vi "HFRR ADV v038 new software.vi"() -> ()   [LabVIEW 2025] (continued)
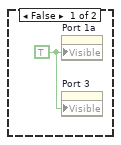
[diagram p5: hidden frame]
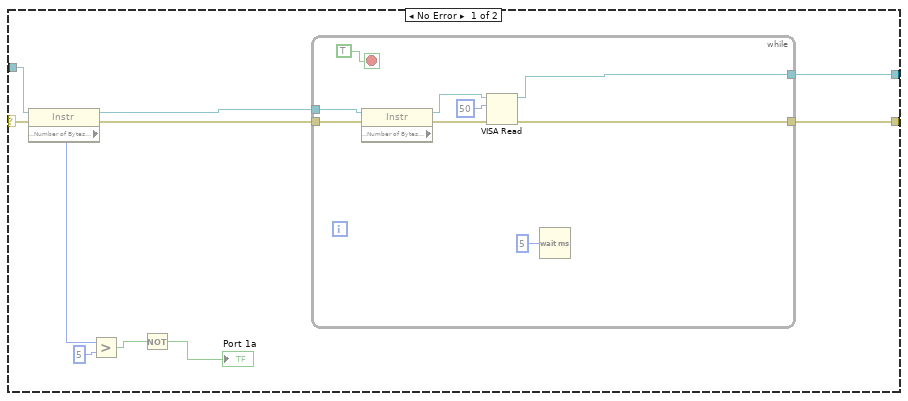
[diagram p6: hidden frame]
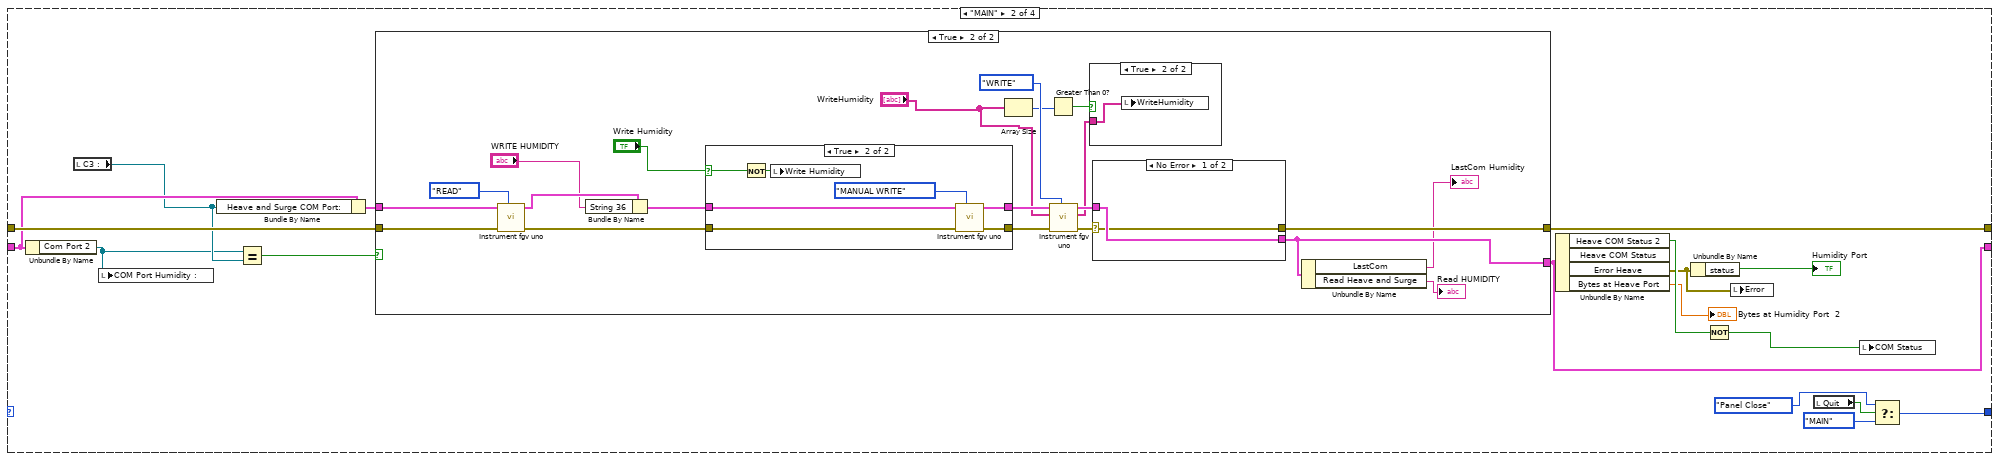
[diagram p9: hidden frame]
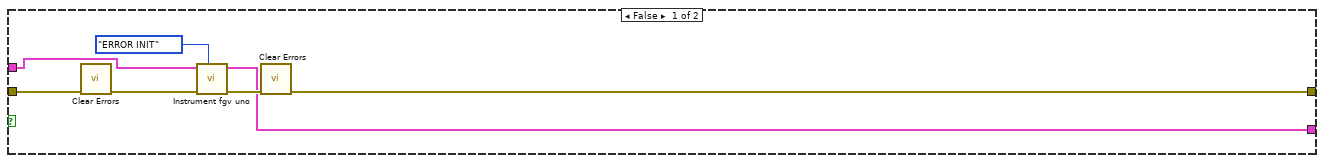
[diagram p10: hidden frame]
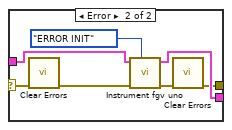
[diagram p12: hidden frame]
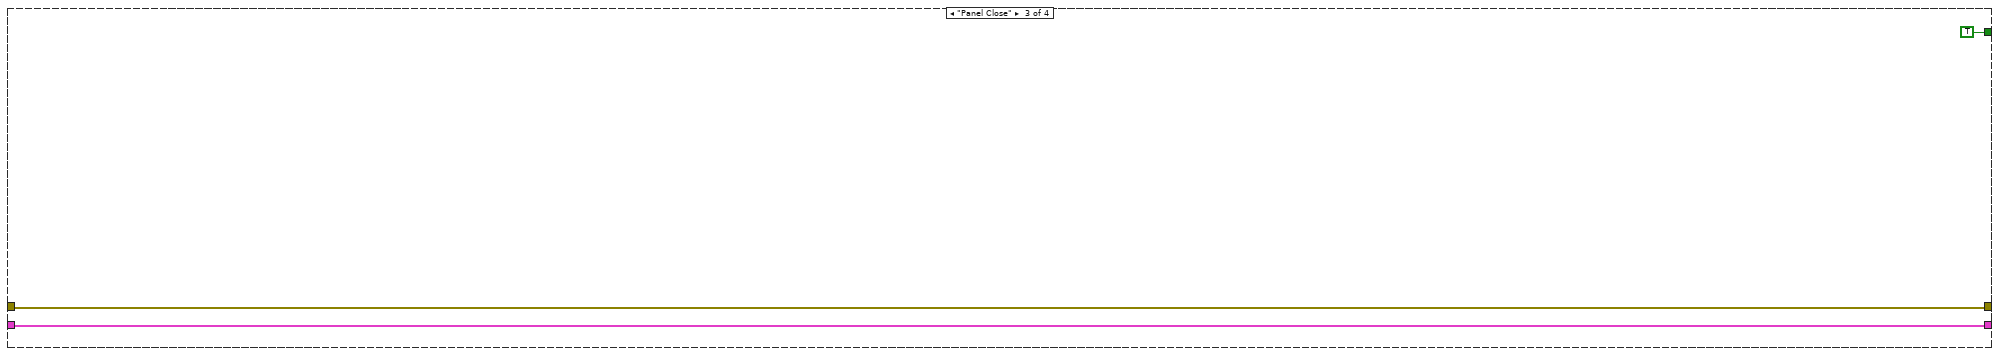
[diagram p14: hidden frame]
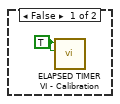
[diagram p18: hidden frame]
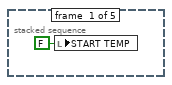
[diagram p20: hidden frame]
        "output Vpp" <- w4065
        n3087 = Number To Fractional String(number=w4065, precision (6)=i16 1) -> (F-format string=w4063:string)  [unwired: 2 in]
        n3088 = Concatenate Strings("DAC;" ("string"), w4063) -> (w4047:string)
        n3089 = local write "Due Write"(w4047) -> ()
        "prev_error" <- w4050
        "integral_accumulator_in" <- w4049
        "prev_vc_cmd" <- w4048
      }
    }
    n3090 = local read "Quit"() -> (w4040:bool)
  }
  n3091 = Or(x=w45, y=w44) -> (x .or. y?=w46:bool)
  n3092 = Or(x=w42, y=w46) -> (x .or. y?=w51:bool)
  n3093 = control-ref of="new picture"() -> ()  [unwired: 1 out]
  n3094 = Or(x=w54, y=w51) -> (x .or. y?=w48:bool)
  n3095 = Or(x=w48, y=w49) -> (x .or. y?=w43:bool)
  n3096 = while {
    tunnel: [w4070] -> w53
    i -> [w4077]
    stop <- w4070 stop-if-true
    n3097 = local read "Quit"() -> (w4070:bool)
    n3098 = Equal To 0?(x=w4077) -> (x = 0?=w4075:bool)
    n3099 = call "Elapsed Time3"("Time Target (s)"=45.0, "Auto Reset"=TRUE) -> ("Time has Elapsed"=w4074:bool)  [unwired: 10 in, 7 out]
    n3100 = Wait (ms)(milliseconds to wait=u32 50) -> ()  [unwired: 1 out]
    n3101 = Or(x=w4074, y=w4075) -> (x .or. y?=w4076:bool)
    n3102 = case shown="True" w4076 {
      frame False {
      }
      frame True {
        n3103 = call <vilib>:"System Exec.vi"("run minimized? (F)"=TRUE, "error in (no error)"="error in (no error)", "command line"="powercfg.exe -change -monitor-timeout-ac 0") -> ("error out"=w4088:errorcluster)  [unwired: 5 in, 3 out]
        n3104 = call <vilib>:"System Exec.vi"("run minimized? (F)"=TRUE, "error in (no error)"=w4088, "command line"="powercfg.exe -change -disk-timeout-ac 0") -> ("error out"=w4087:errorcluster)  [unwired: 5 in, 3 out]
        n3105 = call <vilib>:"System Exec.vi"("run minimized? (F)"=TRUE, "error in (no error)"=w4087, "command line"="powercfg.exe -change -standby-timeout-ac 0") -> ("error out"=w4086:errorcluster)  [unwired: 5 in, 3 out]
        n3106 = call <vilib>:"System Exec.vi"("run minimized? (F)"=TRUE, "error in (no error)"=w4086, "command line"="powercfg.exe -change -hibernate-timeout-ac 0") -> ("error out"=w4085:errorcluster)  [unwired: 5 in, 3 out]
        n3107 = call <vilib>:"Simple Error Handler.vi"("error in (no error)"=w4085) -> ("error out"=w4091:errorcluster)  [unwired: 4 in, 4 out]
        n3108 = call <vilib>:"Clear Errors.vi"("error in (no error)"=w4091) -> ("error out"=→"error out":errorcluster)  [unwired: 5 in, 1 out]
      }
    }
  }
  n3109 = Compound Arithmetic op=OR(w56, w43, w53) -> (w55:bool)
  n3110 = flat-sequence {
    tunnel: w55 -> [_]
    tunnel: [w4093] -> w25
    tunnel: w25 -> [_]
    frame #0 {
      n3111 = call "CLOSE CONNECTION.vi"() -> ("error out"=w4093:errorcluster)  [unwired: 11 in]
    }
    frame #1 {
      n3112 = Quit LabVIEW(quit? (T)=TRUE) -> ()
      n3113 = local write "Quit"(FALSE ("EXIT")) -> ()
    }
  }
  n3114 = property on="Heater Button" class="Bool (strict)"("Visible"=TRUE) -> ()  [unwired: 2 in, 2 out]
  n3115 = while {
    tunnel: [w4100] -> _
    i -> [w4100]
    stop <- w4096 stop-if-true
    # "Langauage selection"
    n3116 = Equal?(x="Lan flag", y=22.0) -> ()  [unwired: 1 out]
    n3117 = disable-structure shown="Disabled" {
      frame Disabled {
        n3118 = stacked-sequence {
          frame #0 {
            n3119 = case shown="\"Russian\"" "Language Selection" {
              tunnel: [0 1] -> w4102
              frame "English", Default {
              }
              frame "Russian" {
              }
            }
            n3120 = for {
              N: 130 -> [_]
              tunnel: "Table" -> [w4111]
              tunnel: w4102 -> [w4110]
              i -> [w4109]
              n3121 = Index Array(array=w4111, index (row)=w4109, index (col)=w4110) -> (element=w4108:string)
              n3122 = case shown="1" w4109 {
                tunnel: w4108 -> [w4112 w4113 _ w4114 w4115 w4116 w4117 w4118 w4119 w4120 w4121 w4122 w4123 w4124 w4125 w4126 w4127 w4128 w4129 w4130 w4131 w4132 w4133 w4134 w4135 w4136 w4137 w4138 w4139 _ _ w4140 w4141 w4142 w4143 w4144 w4145 w4154 w4161 w4168 w4175 w4179 w4182 w4185 w4187 w4189 w4190 w4191 w4192 w4193 w4194 w4195 w4196 w4197 w4198 w4199 w4200 w4201 w4202 w4203 w4204 w4205 w4206 w4207 w4208 w4209 w4210 w4211 w4212 w4213 w4214 w4215 w4216 w4217 w4218 w4219 w4220 w4221 w4222 w4223 w4224 w4225 w4226 w4227 w4228 w4229 w4230 w4231 w4232 w4233 w4234 w4235 w4236 w4237 w4238 w4239 w4240 w4241 w4242 w4243 w4244 w4245 w4246 w4247 w4248 _ w4249 w4250 w4251 w4252 w4253 w4254 w4255 w4256 w4257 w4258 w4259 w4260 w4261 _ w4262 w4263 w4264 w4265 w4266 w4267 _]
                frame 0 {
                  n3123 = local write "S"(w4112) -> ()
                }
                frame 1 {
                  n3124 = local write "S 2"(w4113) -> ()
                }
                frame 2 {
                }
                frame 3 {
                  n3125 = local write "S 4"(w4114) -> ()
                }
                frame 4 {
                  n3126 = property on="FILE" class="Str"("Caption.Text"=w4115) -> ()  [unwired: 2 in, 2 out]
                }
                frame 5 {
                  n3127 = property on="Fuel Discription :" class="Str"("Caption.Text"=w4116) -> ()  [unwired: 2 in, 2 out]
                }
                frame 6 {
                  n3128 = property on="Remarks :" class="Str"("Caption.Text"=w4117) -> ()  [unwired: 2 in, 2 out]
                }
                frame 7 {
                  n3129 = property on="Save & Continue" class="Bool (strict)"("Boolean Text.Text"=w4118) -> ()  [unwired: 2 in, 2 out]
                }
                frame 8 {
                }
                frame 9 {
                  n3130 = property on="Set Hz" class="DigNum (strict)"("Caption.Text"=w4120) -> ()  [unwired: 2 in, 2 out]
                }
                frame 10 {
                }
                frame 11 {
                  n3131 = property on="NORMAL LOAD" class="DigNum (strict)"("Caption.Text"=w4122) -> ()  [unwired: 2 in, 2 out]
                }
                frame 12 {
                }
                frame 13 {
                  n3132 = property on="Set Temp" class="DigNum (strict)"("Caption.Text"=w4124) -> ()  [unwired: 2 in, 2 out]
                }
                frame 14 {
                  n3133 = local write "S 15"(w4125) -> ()
                }
                frame 15 {
                  n3134 = property on="Set Rh" class="DigNum (strict)"("Caption.Text"=w4126) -> ()  [unwired: 2 in, 2 out]
                }
                frame 16 {
                }
                frame 17 {
                  n3135 = local write "S 18"(w4128) -> ()
                }
                frame 18 {
                  "String 17" <- w4129
                }
                frame 19 {
                  n3136 = property on="test time" class="DigNum (strict)"("Caption.Text"=w4130) -> ()  [unwired: 2 in, 2 out]
                }
                frame 20 {
                  "String 18" <- w4131
                  "String 22" <- w4131
                }
                frame 21 {
                  n3137 = property on="Elapsed time" class="DigNum (strict)"("Caption.Text"=w4132) -> ()  [unwired: 2 in, 2 out]
                }
                frame 22 {
                  n3138 = property on="Samplingtime 2" class="DigNum (strict)"("Caption.Text"=w4133) -> ()  [unwired: 2 in, 2 out]
                }
                frame 23 {
                  "String 21" <- w4134
                }
                frame 24 {
                  n3139 = property on="Countdown" class="DigNum (strict)"("Caption.Text"=w4135) -> ()  [unwired: 2 in, 2 out]
                }
                frame 25 {
                  n3140 = property on="Countdown 2" class="DigNum (strict)"("Caption.Text"=w4136) -> ()  [unwired: 2 in, 2 out]
                }
                frame 26 {
                  n3141 = property on="Engage" class="Bool (strict)"("Boolean Text.Text"=w4137) -> ()  [unwired: 2 in, 2 out]
                }
                frame 27 {
                  n3142 = property on="Boolean  4" class="Bool (strict)"("Boolean Text.Text"=w4138) -> ()  [unwired: 2 in, 2 out]
                }
                frame 28 {
                  n3143 = property on="Test \nStatus" class="Bool (strict)"("Boolean Text.Text"=w4139) -> ()  [unwired: 2 in, 2 out]
                }
                frame 29 {
                }
                frame 30 {
                }
                frame 31 {
                }
                frame 32 {
                  n3144 = property on="RSTCOF" class="Bool"("Boolean Text.Text"=w4141) -> ()  [unwired: 2 in, 2 out]
                  n3145 = property on="RST FF" class="Bool"("Boolean Text.Text"=w4141) -> ()  [unwired: 2 in, 2 out]
                  n3146 = property on="RST TEMP" class="Bool"("Boolean Text.Text"=w4141) -> ()  [unwired: 2 in, 2 out]
                  n3147 = property on="RSTV1 3" class="Bool"("Boolean Text.Text"=w4141) -> ()  [unwired: 2 in, 2 out]
                  n3148 = property on="rstv2" class="Bool"("Boolean Text.Text"=w4141) -> ()  [unwired: 2 in, 2 out]
                  n3149 = property on="RSTV1 2" class="Bool"("Boolean Text.Text"=w4141) -> ()  [unwired: 2 in, 2 out]
                  n3150 = property on="RST CP" class="Bool"("Boolean Text.Text"=w4141) -> ()  [unwired: 2 in, 2 out]
                }
                frame 33 {
                  "S 61" <- w4142
                }
                frame 34 {
                  "String 23" <- w4143
                }
                frame 35 {
                  n3151 = property on="Rh Before" class="DigNum (strict)"("Caption.Text"=w4144) -> ()  [unwired: 2 in, 2 out]
                }
                frame 36 {
                  n3152 = Match Pattern(string=w4145, regular expression=",") -> (before substring=→"bs":string, after substring=→"as":string)  [unwired: 1 in, 2 out]
                  n3153 = property on="Rh After" class="DigNum (strict)"("Caption.Text"=w4145) -> ()  [unwired: 2 in, 2 out]
                }
                frame 37 {
                  n3154 = Match Pattern(string=w4154, regular expression=",") -> (before substring=w4153:string, after substring=w4152:string)  [unwired: 1 in, 2 out]
                  "bs" <- w4153
                  "as" <- w4152
                  n3155 = Concatenate Strings(w4153, w4152) -> (w4149:string)
                  n3156 = property on="Humidity before test 2" class="DigNum (strict)"("Caption.Text"=w4149) -> ()  [unwired: 2 in, 2 out]
                  n3157 = Concatenate Strings(w4149, "=" ("string")) -> (w4150:string)
                  n3158 = local write "S 38"(w4150) -> ()
                }
                frame 38 {
                  n3159 = Match Pattern(string=w4161, regular expression=",") -> (before substring=w4160:string, after substring=w4159:string)  [unwired: 1 in, 2 out]
                  "bs" <- w4160
                  "as" <- w4159
                  n3160 = Concatenate Strings(w4160, w4159) -> (w4156:string)
                  n3161 = property on="Humidity after test 2" class="DigNum (strict)"("Caption.Text"=w4156) -> ()  [unwired: 2 in, 2 out]
                  n3162 = Concatenate Strings(w4156, "=" ("string")) -> (w4158:string)
                  n3163 = local write "S 39"(w4158) -> ()
                }
                frame 39 {
                  n3164 = Match Pattern(string=w4168, regular expression=",") -> (before substring=w4167:string, after substring=w4166:string)  [unwired: 1 in, 2 out]
                  "bs" <- w4167
                  "as" <- w4166
                  n3165 = Concatenate Strings(w4167, w4166) -> (w4163:string)
                  n3166 = property on="Temperature before test 2" class="DigNum (strict)"("Caption.Text"=w4163) -> ()  [unwired: 2 in, 2 out]
                  n3167 = Concatenate Strings(w4163, "=" ("string")) -> (→"String 34":string)
                }
                frame 40 {
                  n3168 = Match Pattern(string=w4175, regular expression=",") -> (before substring=w4174:string, after substring=w4173:string)  [unwired: 1 in, 2 out]
                  "bs" <- w4174
                  "as" <- w4173
                  n3169 = Concatenate Strings(w4174, w4173) -> (w4170:string)
                  n3170 = property on="Temperature after test 2" class="DigNum (strict)"("Caption.Text"=w4170) -> ()  [unwired: 2 in, 2 out]
                  n3171 = Concatenate Strings(w4170, "=" ("string")) -> (→"String 35":string)
                  n3172 = property on="Temperature after test" class="DigNum (strict)"("Caption.Text"=w4170) -> ()  [unwired: 2 in, 2 out]
                }
                frame 41 {
                  n3173 = property on="AVP 2" class="DigNum (strict)"("Caption.Text"=w4179) -> ()  [unwired: 2 in, 2 out]
                  n3174 = Concatenate Strings(w4179, "=" ("string")) -> (→"String 36":string)
                }
                frame 42 {
                  n3175 = property on="MWSD 2" class="DigNum (strict)"("Caption.Text"=w4182) -> ()  [unwired: 2 in, 2 out]
                  n3176 = Concatenate Strings(w4182, "=" ("string")) -> (→"String 37":string)
                }
                frame 43 {
                  n3177 = property on="HCF 2" class="DigNum (strict)"("Caption.Text"=w4185) -> ()  [unwired: 2 in, 2 out]
                  n3178 = Concatenate Strings(w4185, "=" ("string")) -> (→"String 38":string)
                }
                frame 44 {
                  n3179 = Concatenate Strings(w4187, "=" ("string")) -> (→"String 39":string)
                  n3180 = property on="WS1.4 2" class="DigNum (strict)"("Caption.Text"=w4187) -> ()  [unwired: 2 in, 2 out]
                }
                frame 45 {
                }
                frame 46 {
                  n3181 = local write "S 47"(w4190) -> ()
                }
                frame 47 {
                  n3182 = local write "S 48"(w4191) -> ()
                }
                frame 48 {
                  n3183 = local write "S 49"(w4192) -> ()
                }
                frame 49 {
                  n3184 = local write "S 50"(w4193) -> ()
                }
                frame 50 {
                  n3185 = local write "S 51"(w4194) -> ()
                }
                frame 51 {
                  n3186 = local write "S 52"(w4195) -> ()
                }
                frame 52 {
                  n3187 = local write "S 53"(w4196) -> ()
                }
                frame 53 {
                  n3188 = local write "S 54"(w4197) -> ()
                }
                frame 54 {
                  n3189 = local write "S 55"(w4198) -> ()
                }
                frame 55 {
                  n3190 = local write "S 56"(w4199) -> ()
                }
                frame 56 {
                  n3191 = local write "S 57"(w4200) -> ()
                }
                frame 57 {
                  n3192 = local write "S 58"(w4201) -> ()
                }
                frame 58 {
                  n3193 = local write "S 59"(w4202) -> ()
                }
                frame 59 {
                  n3194 = local write "S 60"(w4203) -> ()
                }
                frame 60 {
                  n3195 = local write "S 62"(w4204) -> ()
                }
                frame 61 {
                  n3196 = local write "S 63"(w4205) -> ()
                }
                frame 62 {
                  n3197 = local write "S 64"(w4206) -> ()
                }
                frame 63 {
                  n3198 = local write "S 65"(w4207) -> ()
                }
                frame 64 {
                  n3199 = local write "S 66"(w4208) -> ()
                }
                frame 65 {
                  n3200 = local write "S 67"(w4209) -> ()
                }
                frame 66 {
                  n3201 = local write "S 68"(w4210) -> ()
                }
                frame 67 {
                  n3202 = local write "S 69"(w4211) -> ()
                }
                frame 68 {
                  n3203 = local write "S 70"(w4212) -> ()
                }
                frame 69 {
                  n3204 = local write "S 71"(w4213) -> ()
                }
                frame 70 {
                  n3205 = local write "S 72"(w4214) -> ()
                }
                frame 71 {
                  n3206 = local write "S 73"(w4215) -> ()
                }
                frame 72 {
                  n3207 = local write "S 74"(w4216) -> ()
                }
                frame 73 {
                  n3208 = local write "S 75"(w4217) -> ()
                }
                frame 74 {
                  n3209 = local write "S 76"(w4218) -> ()
                }
                frame 75 {
                  n3210 = local write "S 77"(w4219) -> ()
                }
                frame 76 {
                  n3211 = local write "S 78"(w4220) -> ()
                }
                frame 77 {
                  n3212 = local write "S 79"(w4221) -> ()
                }
                frame 79 {
                  n3213 = property on="Sample Temperature ( °C )" class="XYGraph (strict)"("Y Scale.Name Label.Text"=w4222) -> ()  [unwired: 2 in, 2 out]
                }
                frame 80 {
                  n3214 = local write "S 81"(w4223) -> ()
                  n3215 = property on="Humidity ( %RH )" class="XYGraph (strict)"("Y Scale.Name Label.Text"=w4223) -> ()  [unwired: 2 in, 2 out]
                }
                frame 78 {
                  n3216 = property on="Air Temperature  ( °C )" class="XYGraph (strict)"("X Scale.Name Label.Text"=w4224) -> ()  [unwired: 2 in, 2 out]
                  n3217 = property on="Humidity ( %RH )" class="XYGraph (strict)"("X Scale.Name Label.Text"=w4224) -> ()  [unwired: 2 in, 2 out]
                  n3218 = property on="Sample Temperature ( °C )" class="XYGraph (strict)"("X Scale.Name Label.Text"=w4224) -> ()  [unwired: 2 in, 2 out]
                  n3219 = property on="Coefficient Of Friction" class="XYGraph (strict)"("X Scale.Name Label.Text"=w4224) -> ()  [unwired: 2 in, 2 out]
                }
                frame 81 {
                  n3220 = property on="Air Temperature  ( °C )" class="XYGraph (strict)"("Y Scale.Name Label.Text"=w4225) -> ()  [unwired: 2 in, 2 out]
                }
                frame 82 {
                  n3221 = local write "S 84"(w4226) -> ()
                }
                frame 83 {
                  n3222 = local write "S 85"(w4227) -> ()
                }
                frame 84 {
                  n3223 = local write "S 86"(w4228) -> ()
                }
                frame 85 {
                  n3224 = local write "S 87"(w4229) -> ()
                }
                frame 86 {
                  n3225 = local write "S 88"(w4230) -> ()
                }
                frame 87 {
                }
                frame 88 {
                  n3226 = local write "S 90"(w4232) -> ()
                }
                frame 89 {
                  n3227 = local write "S 91"(w4233) -> ()
                }
                frame 90 {
                  n3228 = local write "S 92"(w4234) -> ()
                }
                frame 91 {
                  n3229 = local write "S 93"(w4235) -> ()
                }
                frame 92 {
                  n3230 = local write "S 94"(w4236) -> ()
                }
                frame 93 {
                  n3231 = local write "S 95"(w4237) -> ()
                }
                frame 94 {
                  n3232 = local write "S 96"(w4238) -> ()
                }
                frame 95 {
                  n3233 = local write "S 97"(w4239) -> ()
                }
                frame 96 {
                  n3234 = local write "S 98"(w4240) -> ()
                }
                frame 97 {
                  n3235 = local write "S 99"(w4241) -> ()
                }
                frame 98 {
                  n3236 = local write "S 100"(w4242) -> ()
                }
                frame 99 {
                  n3237 = local write "S 101"(w4243) -> ()
                }
                frame 100 {
                  n3238 = local write "S 102"(w4244) -> ()
                }
                frame 101 {
                  n3239 = local write "S 103"(w4245) -> ()
                }
                frame 102 {
                  n3240 = local write "S 104"(w4246) -> ()
                }
                frame 103 {
                  n3241 = local write "S 105"(w4247) -> ()
                }
                frame 104 {
                  n3242 = local write "S 106"(w4248) -> ()
                }
                frame 105 {
                }
                frame 106 {
                  n3243 = property on="OK Button 17" class="Bool (strict)"("Boolean Text.Text"=w4249) -> ()  [unwired: 2 in, 2 out]
                }
                frame 107 {
                  n3244 = property on="OK Button 16" class="Bool (strict)"("Boolean Text.Text"=w4250) -> ()  [unwired: 2 in, 2 out]
                }
                frame 108 {
                  n3245 = property on="TITTLE" class="Str"("Caption.Text"=w4251) -> ()  [unwired: 2 in, 2 out]
                }
                frame 109 {
                  "String 30" <- w4252
                }
                frame 110 {
                  n3246 = property on="Test Date" class="Str"("Caption.Text"=w4253) -> ()  [unwired: 2 in, 2 out]
                  "String 31" <- w4253
                }
                frame 111 {
                  n3247 = property on="Sample ID" class="Str"("Caption.Text"=w4254) -> ()  [unwired: 2 in, 2 out]
                  "String 32" <- w4254
                }
                frame 112 {
                  n3248 = property on="Tested by" class="Str"("Caption.Text"=w4255) -> ()  [unwired: 2 in, 2 out]
                  "String 33" <- w4255
                }
                frame 113 {
                  n3249 = property on="System Configured Printers 2" class="Arr (strict)"("Caption.Text"=w4256) -> ()  [unwired: 2 in, 2 out]
                }
                frame 114 {
                  n3250 = property on="Selected Printer" class="Str"("Caption.Text"=w4257) -> ()  [unwired: 2 in, 2 out]
                }
                frame 115 {
                  n3251 = property on="Select Printer 3" class="DigNum (strict)"("Caption.Text"=w4258) -> ()  [unwired: 2 in, 2 out]
                }
                frame 116 {
                  n3252 = property on="Print" class="Bool (strict)"("Boolean Text.Text"=w4259) -> ()  [unwired: 2 in, 2 out]
                }
                frame 117 {
                  "String 41" <- w4260
                }
                frame 118 {
                  n3253 = property on="tested by" class="Str"("Caption.Text"=w4261) -> ()  [unwired: 2 in, 2 out]
                }
                frame 119 {
                }
                frame 120 {
                  n3254 = property on="Export" class="Bool (strict)"("Boolean Text.Text"=w4262) -> ()  [unwired: 2 in, 2 out]
                }
                frame 121 {
                }
                frame 122 {
                }
                frame 123 {
                  n3255 = property on="Select File Type" class="Enum (strict)"("Caption.Text"=w4265) -> ()  [unwired: 2 in, 2 out]
                }
                frame 124 {
                  n3256 = property on="s.NO" class="Str"("Caption.Text"=w4266) -> ()  [unwired: 2 in, 2 out]
                  "String 45" <- w4266
                }
                frame 125 {
                  n3257 = property on="trip1 8" class="Bool (strict)"("Boolean Text.Text"=w4267) -> ()  [unwired: 2 in, 2 out]
                }
                frame 126, Default {
                }
              }
            }
          }
          frame #1 {
            w4275 = TRUE ("Visible")
            n3258 = local read "S 91"() -> (w4292:string)
            n3259 = local read "S 90"() -> (w4291:string)
            n3260 = local read "S 88"() -> (w4290:string)
            n3261 = property on="File Path" class="Path"("Caption.Text"=w4291) -> ()  [unwired: 2 in, 2 out]
            n3262 = local read "S 71"() -> (w4285:string)
            n3263 = local read "S 86"() -> (w4287:string)
            n3264 = local read "S 85"() -> (w4288:string)
            n3265 = local read "S 87"() -> (w4286:string)
            n3266 = local read "S 84"() -> (w4289:string)
            n3267 = local read "S 103"() -> (w4274:string)
            n3268 = local read "S 104"() -> (w4273:string)
            n3269 = property on="Password" class="Str"("Caption.Text"=w4288) -> ()  [unwired: 2 in, 2 out]
            n3270 = property on="EDIT" class="Bool (strict)"("Boolean Text.Text"=w4285) -> ()  [unwired: 2 in, 2 out]
            n3271 = property on="SAVE" class="Bool (strict)"("Boolean Text.Text"=w4289) -> ()  [unwired: 2 in, 2 out]
            n3272 = Build Array(w4274, w4273) -> (w4272:string[])
            n3273 = property on="Heater Button" class="Bool (strict)"("Strings [4]"=w4272) -> ()  [unwired: 2 in, 2 out]
            n3274 = local read "S 92"() -> (w4284:string)
            n3275 = local read "S 93"() -> (w4283:string)
            n3276 = local read "S 105"() -> (w4270:string)
            n3277 = local read "S 106"() -> (w4269:string)
            n3278 = Build Array(w4284, w4283) -> ()  [unwired: 1 out]
            n3279 = Build Array(w4270, w4269) -> (w4271:string[])
            n3280 = local read "S 95"() -> (w4281:string)
            n3281 = local read "S 94"() -> (w4282:string)
            n3282 = local read "bs"() -> (w4297:string)
            n3283 = local read "as"() -> (w4298:string)
            n3284 = property on="Humidity" class="Bool (strict)"("Strings [4]"=w4271) -> ()  [unwired: 2 in, 2 out]
            n3285 = Concatenate Strings(w4297, "\r", w4298) -> ()  [unwired: 1 out]
            n3286 = property on="Rh After" class="DigNum (strict)"("Caption.Size to Text?"=TRUE ("Caption.Size to Text")) -> ()  [unwired: 2 in, 2 out]
            n3287 = local read "S 48"() -> (w4321:string)
            n3288 = local read "S 50"() -> (w4319:string)
            n3289 = local read "S 51"() -> (w4318:string)
            n3290 = local read "S 49"() -> (w4320:string)
            n3291 = local read "S 52"() -> (w4317:string)
            n3292 = local read "as"() -> (w4302:string)
            n3293 = local read "bs"() -> (w4303:string)
            n3294 = local read "S 56"() -> (w4316:string)
            n3295 = local read "S 57"() -> (w4315:string)
            n3296 = local read "S 58"() -> (w4314:string)
            n3297 = local read "S 59"() -> (w4313:string)
            n3298 = property on="OPEN" class="Bool (strict)"("Boolean Text.Text"=w4317) -> ()  [unwired: 2 in, 2 out]
            n3299 = property on="OPEN 1" class="Bool (strict)"("Boolean Text.Text"=w4321) -> ()  [unwired: 2 in, 2 out]
            n3300 = property on="OPEN 2" class="Bool (strict)"("Boolean Text.Text"=w4320) -> ()  [unwired: 2 in, 2 out]
            n3301 = property on="OPEN 3" class="Bool (strict)"("Boolean Text.Text"=w4319) -> ()  [unwired: 2 in, 2 out]
            n3302 = property on="OPEN 4" class="Bool (strict)"("Boolean Text.Text"=w4318) -> ()  [unwired: 2 in, 2 out]
            n3303 = Concatenate Strings(w4303, "\r", w4302) -> ()  [unwired: 1 out]
            n3304 = local read "S 102"() -> (w4276:string)
            n3305 = property on="КОФ1" class="DigNum (strict)"("Caption.Text"=w4316) -> ()  [unwired: 2 in, 2 out]
            n3306 = local read "S 98"() -> (w4280:string)
            n3307 = local read "S 99"() -> (w4279:string)
            n3308 = local read "S 100"() -> (w4278:string)
            n3309 = local read "S 101"() -> (w4277:string)
            n3310 = property on="КОФ2" class="DigNum (strict)"("Caption.Text"=w4315) -> ()  [unwired: 2 in, 2 out]
            n3311 = property on="КОФ3" class="DigNum (strict)"("Caption.Text"=w4314) -> ()  [unwired: 2 in, 2 out]
            n3312 = property on="КОФ4" class="DigNum (strict)"("Caption.Text"=w4313) -> ()  [unwired: 2 in, 2 out]
            n3313 = local read "bs"() -> (w4301:string)
            n3314 = local read "as"() -> (w4300:string)
            n3315 = local read "S 60"() -> (w4312:string)
            n3316 = local read "S 54"() -> (w4322:string)
            n3317 = Concatenate Strings(w4301, "\r", w4300) -> ()  [unwired: 1 out]
            n3318 = Concatenate Strings(w4322, w4312) -> ()  [unwired: 1 out]
            n3319 = local read "S 77"() -> (→"String 43":string)
            n3320 = local read "S 76"() -> (w4295:string)
            n3321 = local read "S 78"() -> (w4294:string)
            n3322 = local read "S 71"() -> (w4306:string)
            n3323 = local read "S 66"() -> (w4311:string)
            n3324 = local read "S 67"() -> (w4310:string)
            n3325 = local read "S 68"() -> (w4309:string)
            n3326 = local read "S 69"() -> (w4308:string)
            n3327 = local read "S 70"() -> (w4307:string)
            n3328 = property on="AIR TEMP" class="DigNum (strict)"("Caption.Text"=w4294) -> ()  [unwired: 2 in, 2 out]
            n3329 = property on="Set Strk" class="DigNum (strict)"("Caption.Text"=w4295) -> ()  [unwired: 2 in, 2 out]
            n3330 = property on="SPEED OUT:" class="DigNum (strict)"("Caption.Text"=w4309) -> ()  [unwired: 2 in, 2 out]
            n3331 = property on="EDIT" class="Bool (strict)"("Boolean Text.Text"=w4306) -> ()  [unwired: 2 in, 2 out]
            n3332 = local read "S 79"() -> (w4293:string)
          }
          frame #2 {
          }
        }
        n3333 = local write "Lan flag"(10.0 ("Lan flag")) -> ()
      }
      frame Enabled {
      }
    }
    n3334 = Wait (ms)(milliseconds to wait=u32 2000) -> ()  [unwired: 1 out]
    n3335 = local read "Quit"() -> (w4096:bool)
  }
  n3336 = while {
    shift-right: [w4328] -> _
    shift-left: _ -> [w4329]
    shift-right: [w4326] -> _
    shift-left: T18 {"Read Heave and Surge"="", "Bytes at Heave Port"=0.0, "Heave and Surge COM Port:"="COM9", "Com Port 2"="COM7", "Residual Due"="", "Heave COM Status 2"=TRUE, "Heave COM Status"=TRUE, "Port 2"=TRUE, "Sway PPR"=6400.0, "Surge PPR"=6400.0, "Heave PPR"=6400.0, "Sway Pitch"=2.0, "Surge Pitch"=3.0, "Heave Pitch"=4.0, "Sway Pulses/mm"=320.0, "Surge Pulses/mm"=1600.0, "Heave Pulses/mm"=1600.0, "inner loop"=0.0, "Read Heave and Surge 2"="", "String 36"="", "Write S"=FALSE, "WriteCC1"=[""], "Heave COM Loop"=0, "LastCom"="", "EXIT"=FALSE, "Error Heave"={"status"=TRUE, "code"=-1073807343, "source"=""}} -> [w4325]
    shift-right: [w4323] -> _
    shift-left: enum16{"init", "MAIN", "Panel Close"}."init" -> [w4324]
    stop <- w4327 stop-if-true
    # "HUMIDITY LOOP LOGIC"
    n3337 = case shown="\"init\"" w4324 {
      tunnel: w4329 -> [w4343 w4362 w4417 w4419]
      tunnel: [w4338 w4366 w4417 w4419] -> w4328
      tunnel: [_ _ TRUE _] -> w4327
      tunnel: [w4335 w4364 w4415 w4418] -> w4326
      tunnel: w4325 -> [w4340 w4361 w4415 w4418]
      tunnel: [enum16{"init", "MAIN", "Panel Close"}."MAIN" w4356 _ _] -> w4323
      frame "init" {
        n3338 = local read "C3 :"() -> (w4330:refnum<visa-resource-name>)
        n3339 = Bundle By Name(cluster=w4340, "Heave and Surge COM Port:"=w4330) -> (w4339:T18)
        n3340 = call "Instrument fgv uno.vi"("Enum"=T31."INIT", "error in (no error) 2"=w4343, "INPUT"=w4339) -> ("error"=w4341:errorcluster, "output"=w4337:T18)  [unwired: 6 in, 1 out]
        n3341 = case shown="Error" w4341 {
          selector: w4341 -> [w4345 _]
          tunnel: [w4345 w4349] -> w4338
          tunnel: w4337 -> [w4344 w4347]
          tunnel: [w4344 w4346] -> w4336
          frame No Error {
          }
          frame Error {
            n3342 = call "Instrument fgv uno.vi"("Enum"=T31."ERROR INIT", "INPUT"=w4347) -> ("error"=w4350:errorcluster, "output"=w4346:T18)  [unwired: 7 in, 1 out]
            n3343 = call <vilib>:"Clear Errors.vi"("error in (no error)"=w4350) -> ("error out"=w4349:errorcluster)  [unwired: 5 in, 1 out]
          }
        }
        n3344 = local read "LastCom Humidity"() -> (w4333:string)
        n3345 = Unbundle By Name(w4336) -> ("Heave COM Status 2"=→"COM Status":bool, "Error Heave"=→"Error":errorcluster)  [unwired: 1 out]
        n3346 = Bundle By Name(cluster=w4336, "LastCom"=w4333) -> (w4335:T18)
      }
      frame "MAIN" {
        n3347 = Unbundle By Name(w4361) -> ("Com Port 2"=w4351:refnum<visa-resource-name>)
        n3348 = local read "C3 :"() -> (w4352:refnum<visa-resource-name>)
        n3349 = local write "COM Port Humidity :"(w4351) -> ()
        n3350 = Bundle By Name(cluster=w4361, "Heave and Surge COM Port:"=w4352) -> (w4360:T18)
        n3351 = Equal?(x=w4351, y=w4352) -> (x = y?=w4367:bool)
        n3352 = case shown="True" w4367 {
          tunnel: [w4371 w4388] -> w4366
          tunnel: w4362 -> [w4372 w4394]
          tunnel: w4360 -> [w4370 w4392]
          tunnel: [w4369 w4387] -> w4364
          frame False {
            n3353 = call <vilib>:"Clear Errors.vi"("error in (no error)"=w4372) -> ("error out"=w4368:errorcluster)  [unwired: 5 in, 1 out]
            n3354 = call "Instrument fgv uno.vi"("Enum"=T31."ERROR INIT", "error in (no error) 2"=w4368, "INPUT"=w4370) -> ("error"=w4374:errorcluster, "output"=w4369:T18)  [unwired: 6 in, 1 out]
            n3355 = call <vilib>:"Clear Errors.vi"("error in (no error)"=w4374) -> ("error out"=w4371:errorcluster)  [unwired: 5 in, 1 out]
          }
          frame True {
            n3356 = call "Instrument fgv uno.vi"("Enum"=T31."READ", "error in (no error) 2"=w4394, "INPUT"=w4392) -> ("error"=w4393:errorcluster, "output"=w4386:T18)  [unwired: 6 in, 1 out]
            n3357 = Bundle By Name(cluster=w4386, "String 36"="WRITE HUMIDITY") -> (w4385:T18)
            n3358 = case shown="True" "Write Humidity" {
              selector: "Write Humidity" -> [_ w4414]
              tunnel: w4393 -> [w4407 w4413]
              tunnel: [w4407 w4412] -> w4383
              tunnel: w4385 -> [w4406 w4410]
              tunnel: [w4406 w4409] -> w4382
              frame False {
              }
              frame True {
                n3359 = Not(x=w4414) -> (.not. x?=w4408:bool)
                n3360 = local write "Write Humidity"(w4408) -> ()
                n3361 = call "Instrument fgv uno.vi"("Enum"=T31."MANUAL WRITE", "error in (no error) 2"=w4413, "INPUT"=w4410) -> ("error"=w4412:errorcluster, "output"=w4409:T18)  [unwired: 6 in, 1 out]
              }
            }
            n3362 = Array Size(array="WriteHumidity") -> (size(s)=w4380:i32)
            n3363 = Greater Than 0?(x=w4380) -> (x > 0?=w4379:bool)
            n3364 = call "Instrument fgv uno.vi"("Enum"=T31."WRITE", "error in (no error) 2"=w4383, "WriteCC1"="WriteHumidity", "INPUT"=w4382) -> ("error"=w4390:errorcluster, "WriteCC1 2"=w4381:string[], "output"=w4389:T18)  [unwired: 5 in]
            n3365 = case shown="True" w4379 {
              tunnel: w4381 -> [_ w4396]
              frame False {
              }
              frame True {
                n3366 = local write "WriteHumidity"(w4396) -> ()
              }
            }
            n3367 = case shown="No Error" w4390 {
              selector: w4390 -> [w4397 w4400]
              tunnel: w4389 -> [w4398 w4405]
              tunnel: [w4398 w4404] -> w4387
              tunnel: [w4397 w4402] -> w4388
              frame No Error {
              }
              frame Error {
                n3368 = call <vilib>:"Clear Errors.vi"("error in (no error)"=w4400) -> ("error out"=w4399:errorcluster)  [unwired: 5 in, 1 out]
                n3369 = call "Instrument fgv uno.vi"("Enum"=T31."ERROR INIT", "error in (no error) 2"=w4399, "INPUT"=w4405) -> ("error"=w4403:errorcluster, "output"=w4404:T18)  [unwired: 6 in, 1 out]
                n3370 = call <vilib>:"Clear Errors.vi"("error in (no error)"=w4403) -> ("error out"=w4402:errorcluster)  [unwired: 5 in, 1 out]
              }
            }
            n3371 = Unbundle By Name(w4387) -> ("LastCom"=→"LastCom Humidity":string, "Read Heave and Surge"=→"Read HUMIDITY":string)
          }
        }
        n3372 = Unbundle By Name(w4364) -> ("Heave COM Status 2"=w4365:bool, "Error Heave"=w4353:errorcluster, "Bytes at Heave Port"=→"Bytes at Humidity Port  2":dbl)  [unwired: 1 out]
        n3373 = Unbundle By Name(w4353) -> ("status"=→"Humidity Port":bool)
        n3374 = Not(x=w4365) -> (.not. x?=w4354:bool)
        n3375 = local write "Error"(w4353) -> ()
        n3376 = local read "Quit"() -> (w4357:bool)
        n3377 = local write "COM Status"(w4354) -> ()
        n3378 = Select(t=enum16{"init", "MAIN", "Panel Close"}."Panel Close", s=w4357, f=enum16{"init", "MAIN", "Panel Close"}."MAIN") -> (s? t:f=w4356:enum16{"init", "MAIN", "Panel Close"})
      }
      frame "Panel Close" {
      }
      frame Default {
      }
    }
  }
  n3379 = while {
    stop <- w4422 stop-if-true
    n3380 = call <vilib>:"High Resolution Polling Wait.vi"("seconds to wait"=0.05) -> ()  [unwired: 10 in, 1 out]
    n3381 = disable-structure shown="Disabled" {
      disable-tunnel: [_ w4453] -> w4420
      frame Disabled {
        n3382 = local read "Read HUMIDITY"() -> (w4423:string)
        n3383 = Spreadsheet String To Array(delimiter (Tab)=",", format string="", spreadsheet string=w4423, array type (2D Dbl)=string[] []) -> (array=w4442:string[])
        n3384 = for {
          tunnel: w4442 -> [w4451] mode=indexing
          tunnel: string[] ["STATE;", "SET;", "RH;", "T;", "AMB_RH;", "AMB_T;", "PUMP;", "FAN_IN;", "FAN_OUT;", "DEHUM;", "CURRENT;", "STALL;"] -> [w4450] mode=indexing
          tunnel: [w4449] -> w4441 mode=indexing
          n3385 = Match Pattern(string=w4451, regular expression=w4450) -> (after substring=w4449:string)  [unwired: 1 in, 3 out]
        }
        n3386 = Index Array(array=w4441) -> (element #1=→"STATE :":string, element #2=→"SET :":string, element #3=w4431:string, element #4=→"T :":string, element #5=w4429:string, element #6=→"AMB_T :":string, element #7=→"PUMP :":string, element #8=→"FAN_IN :":string, element #9=→"FAN_OUT :":string, element #10=→"DEHUM :":string, element #11=→"CURRENT :":string, element #12=→"STALL :":string)  [unwired: 12 in]
        "RH :" <- w4431
        "AMB_RH :" <- w4429
        n3387 = Fract/Exp String To Number(string=w4431) -> (number=w4424:dbl)  [unwired: 3 in, 1 out]
        n3388 = Fract/Exp String To Number(string=w4429) -> (number=w4428:dbl)  [unwired: 3 in, 1 out]
        n3389 = local write "Ambient Humidity :"(w4428) -> ()
        n3390 = Equal?(x=w4424, y=0.0) -> (x = y?=w4426:bool)
        n3391 = case shown="True" w4426 {
          tunnel: [w4447 w4448] -> w4425
          tunnel: w4424 -> [w4447 _]
          frame False {
            (unwired) 0.0
            "Humidity temp" <- w4447
          }
          frame True {
            n3392 = local read "Humidity temp"() -> (w4448:dbl)
          }
        }
        "RH Numeric:" <- w4425
      }
      frame Enabled {
        n3393 = local read "Read HUMIDITY"() -> (w4474:string)
        n3394 = Spreadsheet String To Array(delimiter (Tab)=",", format string="", spreadsheet string=w4474, array type (2D Dbl)=dbl[] []) -> (array=w4470:dbl[])
        n3395 = Index Array(array=w4470) -> (element #1=→"STATE :":dbl, element #2=→"SET :":dbl, element #3=w4455:dbl, element #4=→"RH :":dbl, element #5=→"T :":dbl, element #6=→"AMB_RH :":dbl, element #7=→"AMB_T :":dbl, element #8=→"PUMP :":dbl, element #9=→"FAN_IN :":dbl, element #10=→"FAN_OUT :":dbl, element #11=→"DEHUM :":dbl, element #12=→"CURRENT :":dbl, element #13=→"STALL":dbl)  [unwired: 13 in]
        "RH Numeric:" <- w4455
        n3396 = Equal?(x=w4455, y=0.0) -> (x = y?=w4458:bool)
        n3397 = case shown="False" w4458 {
          tunnel: [w4475 w4476] -> w4454
          tunnel: w4455 -> [w4475 _]
          frame False {
            "Humidity temp 2" <- w4475
          }
          frame True {
            n3398 = local read "Humidity temp 2"() -> (w4476:dbl)
          }
        }
        n3399 = call <vilib>:"Median Filter PtByPt.vi"("rank"=2, "x"=w4454) -> ("Filtered x"=w4453:dbl)  [unwired: 2 in, 1 out]
      }
    }
    n3400 = local write "RH Numeric:"(w4420) -> ()
    n3401 = local read "Quit"() -> (w4422:bool)
  }
  n3402 = while {
    shift-right: [w4482] -> _
    shift-left: _ -> [w4483]
    shift-right: [w4480] -> _
    shift-left: T20 {"Read Uno"="", "Bytes at Heave Port"=0.0, "UNO COM Port:"="COM9", "UNO COM Port: 2"="COM7", "Residual Due"="", "UNO COM Status 2"=TRUE, "UNO COM Status"=TRUE, "Port 2"=TRUE, "Sway PPR"=6400.0, "Surge PPR"=6400.0, "Heave PPR"=6400.0, "Sway Pitch"=2.0, "Surge Pitch"=3.0, "Heave Pitch"=4.0, "Sway Pulses/mm"=320.0, "Surge Pulses/mm"=1600.0, "Heave Pulses/mm"=1600.0, "inner loop"=0.0, "Read Heave and Surge 2"="", "String 36"="", "Write S"=FALSE, "WriteCC1"=[""], "Heave COM Loop"=0, "LastCom"="", "EXIT"=FALSE, "Error Heave"={"status"=TRUE, "code"=-1073807343, "source"=""}} -> [w4479]
    shift-right: [w4477] -> _
    shift-left: enum16{"init", "MAIN", "Panel Close"}."init" -> [w4478]
    stop <- w4481 stop-if-true
    # "UNO CODE LOGIC"
    n3403 = case shown="\"MAIN\"" w4478 {
      tunnel: w4483 -> [w4497 w4516 w4572 w4574]
      tunnel: [w4492 w4521 w4572 w4574] -> w4482
      tunnel: [_ _ TRUE _] -> w4481
      tunnel: [w4488 w4519 w4570 w4573] -> w4480
      tunnel: w4479 -> [w4494 w4515 w4570 w4573]
      tunnel: [enum16{"init", "MAIN", "Panel Close"}."MAIN" w4510 _ _] -> w4477
      frame "init" {
        n3404 = local read "Com Port 1"() -> (w4484:refnum<visa-resource-name>)
        n3405 = Bundle By Name(cluster=w4494, "UNO COM Port:"=w4484) -> (w4493:T20)
        n3406 = call "Instrument fgv.vi"("Enum"=T31."INIT", "error in (no error) 2"=w4497, "INPUT"=w4493) -> ("error"=w4495:errorcluster, "output"=w4491:T18)  [unwired: 6 in, 1 out]
        n3407 = case shown="Error" w4495 {
          selector: w4495 -> [w4499 _]
          tunnel: [w4499 w4503] -> w4492
          tunnel: w4491 -> [w4498 w4501]
          tunnel: [w4498 w4500] -> w4489
          frame No Error {
          }
          frame Error {
            n3408 = call "Instrument fgv.vi"("Enum"=T31."ERROR INIT", "INPUT"=w4501) -> ("error"=w4504:errorcluster, "output"=w4500:T18)  [unwired: 7 in, 1 out]
            n3409 = call <vilib>:"Clear Errors.vi"("error in (no error)"=w4504) -> ("error out"=w4503:errorcluster)  [unwired: 5 in, 1 out]
          }
        }
        n3410 = local read "LastCom UNO"() -> (w4486:string)
        n3411 = Unbundle By Name(w4489) -> ("Heave COM Status 2"=→"Instrument Status":bool, "Error Heave"=→"Error  2":errorcluster)  [unwired: 1 out]
        n3412 = Bundle By Name(cluster=w4489, "LastCom"=w4486) -> (w4488:T18)
      }
      frame "MAIN" {
        n3413 = Unbundle By Name(w4515) -> ("UNO COM Port: 2"=w4505:refnum<visa-resource-name>)
        n3414 = local read "Com Port 1"() -> (w4506:refnum<visa-resource-name>)
        n3415 = local write "COM Port UNO :"(w4505) -> ()
        n3416 = Equal?(x=w4505, y=w4506) -> (x = y?=w4522:bool)
        n3417 = Bundle By Name(cluster=w4515, "UNO COM Port:"=w4506) -> (w4514:T20)
        n3418 = case shown="True" w4522 {
          tunnel: [w4526 w4543] -> w4521
          tunnel: w4516 -> [w4527 w4549]
          tunnel: w4514 -> [w4525 w4547]
          tunnel: [w4524 w4542] -> w4519
          frame False {
            n3419 = call <vilib>:"Clear Errors.vi"("error in (no error)"=w4527) -> ("error out"=w4523:errorcluster)  [unwired: 5 in, 1 out]
            n3420 = call "Instrument fgv.vi"("Enum"=T31."ERROR INIT", "error in (no error) 2"=w4523, "INPUT"=w4525) -> ("error"=w4529:errorcluster, "output"=w4524:T18)  [unwired: 6 in, 1 out]
            n3421 = call <vilib>:"Clear Errors.vi"("error in (no error)"=w4529) -> ("error out"=w4526:errorcluster)  [unwired: 5 in, 1 out]
          }
          frame True {
            n3422 = call "Instrument fgv.vi"("Enum"=T31."READ", "error in (no error) 2"=w4549, "INPUT"=w4547) -> ("error"=w4548:errorcluster, "output"=w4541:T18)  [unwired: 6 in, 1 out]
            n3423 = Bundle By Name(cluster=w4541, "String 36"="WRITE UNO") -> (w4540:T18)
            n3424 = case shown="True" "Write" {
              selector: "Write" -> [_ w4564]
              tunnel: w4548 -> [w4562 w4569]
              tunnel: [w4562 w4568] -> w4538
              tunnel: w4540 -> [w4561 w4566]
              tunnel: [w4561 w4565] -> w4537
              frame False {
              }
              frame True {
                n3425 = Not(x=w4564) -> (.not. x?=w4563:bool)
                n3426 = local write "Write"(w4563) -> ()
                n3427 = call "Instrument fgv.vi"("Enum"=T31."MANUAL WRITE", "error in (no error) 2"=w4569, "INPUT"=w4566) -> ("error"=w4568:errorcluster, "output"=w4565:T18)  [unwired: 6 in, 1 out]
              }
            }
            n3428 = Array Size(array="Write UNO") -> (size(s)=w4535:i32)
            n3429 = Greater Than 0?(x=w4535) -> (x > 0?=w4534:bool)
            n3430 = call "Instrument fgv.vi"("Enum"=T31."WRITE", "error in (no error) 2"=w4538, "WriteCC1"="Write UNO", "INPUT"=w4537) -> ("error"=w4545:errorcluster, "WriteCC1 2"=w4536:string[], "output"=w4544:T18)  [unwired: 5 in]
            n3431 = case shown="True" w4534 {
              tunnel: w4536 -> [_ w4551]
              frame False {
              }
              frame True {
                n3432 = local write "Write UNO"(w4551) -> ()
              }
            }
            n3433 = case shown="Error" w4545 {
              selector: w4545 -> [w4552 w4555]
              tunnel: w4544 -> [w4553 w4560]
              tunnel: [w4553 w4559] -> w4542
              tunnel: [w4552 w4557] -> w4543
              frame No Error {
              }
              frame Error {
                n3434 = call <vilib>:"Clear Errors.vi"("error in (no error)"=w4555) -> ("error out"=w4554:errorcluster)  [unwired: 5 in, 1 out]
                n3435 = call "Instrument fgv.vi"("Enum"=T31."ERROR INIT", "error in (no error) 2"=w4554, "INPUT"=w4560) -> ("error"=w4558:errorcluster, "output"=w4559:T18)  [unwired: 6 in, 1 out]
                n3436 = call <vilib>:"Clear Errors.vi"("error in (no error)"=w4558) -> ("error out"=w4557:errorcluster)  [unwired: 5 in, 1 out]
              }
            }
            n3437 = Unbundle By Name(w4542) -> ("LastCom"=→"LastCom UNO":string, "Read Heave and Surge"=→"Read UNO":string)
          }
        }
        n3438 = Unbundle By Name(w4519) -> ("Heave COM Status 2"=w4520:bool, "Heave COM Status"=w4509:bool, "Error Heave"=w4507:errorcluster, "Bytes at Heave Port"=→"Bytes at Humidity Port":dbl)
        n3439 = Not(x=w4509) -> (.not. x?=w4517:bool)
        n3440 = Not(x=w4520) -> (.not. x?=w4508:bool)
        n3441 = local write "Instrument Status"(w4517) -> ()
        n3442 = local write "Error  2"(w4507) -> ()
        n3443 = local write "Port 1a"(w4509) -> ()
        n3444 = local read "Quit"() -> (w4511:bool)
        n3445 = local write "COM Status"(w4508) -> ()
        n3446 = Select(t=enum16{"init", "MAIN", "Panel Close"}."Panel Close", s=w4511, f=enum16{"init", "MAIN", "Panel Close"}."MAIN") -> (s? t:f=w4510:enum16{"init", "MAIN", "Panel Close"})
      }
      frame "Panel Close" {
      }
      frame Default {
      }
    }
  }
